vi "TabVisibility.vi"(1 "Page Visible":bool, 2 "array":refnum<vi>[](array[refnum]), 3 "MyfinalExpGraphCont":T1(tab)) -> ()   [LabVIEW 2019]
uses:
  C:/Users/manip/Documents/Controle_Manip_2020/Thorlabs.MotionControl.Controls.dll
  Thorlabs.MotionControl.Controls.dll
  C:/Users/manip/Documents/Controle_Manip_2020/Thorlabs.MotionControl.KCube.SolenoidCLI.dll
  Thorlabs.MotionControl.KCube.SolenoidCLI.dll
  C:/Users/manip/Documents/Controle_Manip_2020/Thorlabs.MotionControl.KCube.PiezoCLI.dll
  Thorlabs.MotionControl.KCube.PiezoCLI.dll
  C:/Program Files/Thorlabs/Scientific Imaging/DCx Camera Support/Develop/DotNet/uc480DotNet.dll
  Program Files/Thorlabs/Scientific Imaging/DCx Camera Support/Develop/DotNet/uc480DotNet.dll
  Light Field/lightfield-automation-labview/LightField Automation.lvclass
  Controls/Control 1.ctl
panel:
  out "Duration 2":dbl caption="s"
  in  "Acquire N: N 2":dbl=10.0 caption="N"
  in  "Acquire Time Trace 2":bool caption="Acquire N"
  in  "CCD 1D Spectrum Main  Cursor2WL 2 Mono 4":bool caption="CCD 1D Spectrum Main  Cursor2WL"
  in  "CCD 1D Spectrum Main  Cursor2WL 1 Mono 4":bool caption="CCD 1D Spectrum Main  Cursor2WL"
  in  "CCD 1D Spectrum Main  Cursor2WL 2 Mono 3":bool caption="CCD 1D Spectrum Main  Cursor2WL"
  in  "CCD 1D Spectrum Main  Cursor2WL 1 Mono 3":bool caption="CCD 1D Spectrum Main  Cursor2WL"
  out "CCD 1D Spectrum Main Cursor 1 nm 2":dbl caption="nm"
  out "CCD 1D Spectrum Main Cursor 2 nm 2":dbl caption="nm"
  in  "Full scale 2":bool
  in  "Acquire Continuous Spectrum 2":bool
  in  "Acquire Spectrum 2":bool
  out "CCD 2D Image Main 2":dbl[][](graph)
  in  "Save Spectrum N 2":bool
  in  "Save Spectrum 2":bool
  out "CCD 1D Spectrum Main 2":T2
  in  "Stop continuous 2":bool
  out "CCD 1D Spectrum Main Energy Scale 2":cluster{dbl[], dbl[]}(graph)
  out "CCD 1D Spectrum Main Cursor 4":dbl caption="eV" format="%#_6p"
  out "CCD 1D Spectrum Main Cursor 3":dbl caption="eV" format="%#_6p"
  out "CCD 1D Spectrum Main deltaE 2":dbl caption="eV" format="%#_3p"
  out "CCD 1D Spectrum Main deltanm 2":dbl caption="m" format="%#_3p"
  in  "Scan FSM Set as Center 2":bool
  in  "Scan FSM Go to Cursor 2":bool
  out "XY Intensity Map 2":dbl[][](graph)
  out "CCD 2D Image XY Map 2":dbl[][](graph)
  out "CCD 1D Spectrum XY Map 2":cluster{dbl[], dbl[]}(graph)
  out "CCD 1D XY Map Spectrum Main Energy Scale 2":cluster{dbl[], dbl[]}(graph)
  in  "NewDot 2":bool caption="NewDot?"
  out "ExportMapPosition? 2":bool caption="Export NC Pos in Map Image?"
  out "Polarisation 2D Image 2":dbl[][](graph)
  out "Polarisation 1D Spectrum 2":cluster{dbl[], dbl[]}(graph) caption="360.0°"
  out "Polarisation 1D Spectrum Energy Scale 2":cluster{dbl[], dbl[]}(graph)
  out "Contrast 2":dbl format="%#_3g"
  out "Contrast Oscillations 2":cluster{dbl[], dbl[]}(graph)
  out "Contrast 1D Spectrum 2":cluster{dbl[], dbl[]}(graph) caption="52924"
  in  "Cursor controls 2":bool
  out "Contrast 1D Spectrum from Cursors 2":cluster{dbl[], dbl[]}(graph) caption="2708"
  in  "Spectrum Custom Continuous Mode 2":u16(ring)=1 caption="Detector(s)" items=["PD", "APD 1", "APD 2", "APD 1+2"]
  in  "Stop PD 2":bool
  in  "Acquire PD 2":bool
  out "PD 1D Spectrum 2":dbl[][](graph)
  in  "PH_SyncDiv 2":enum16{"1", "2", "4", "8"}(ring) caption="SyncDiv"
  in  "PH_CFD0 level 2":i32=50 caption="CFD0" min=0 max=100
  in  "PH_CFD0 zero X 2":i32=10 caption="CFD0 ZeroX"
  in  "PH_CFD1 level 2":i32=50 caption="CFD1" min=0 max=100
  in  "PH_CFD1 zero X 2":i32=10 caption="CFD1 Zero X"
  in  "PH_Range No. 2":i32 caption="Range No."
  in  "V2um 2":dbl=10.0
  in  "Conv/Energy (eV) 2":dbl caption="Energy :" format="%#_6p"
  in  "Conv/Wavelength (nm) 2":dbl caption="Wavelength :"
  in  "Conv/Wavenumber (m-1) 2":dbl caption="Wavenumber :"
  in  "Conv/Time (s) 2":dbl caption="Time :" format="%#_6p"
  in  "ChangeSample 2":bool
  in  "SampleGoal 2":string
  in  "Write to Markdown? 2":bool
  in  "Synthesis/Solvent 2":string(combo)="tol"
  in  "Synthesis/Polymer 2":string(combo)="PS"
  in  "Synthesis/DilutionPolyRatio 2":dbl=1.5
  in  "SampleOf 2":string(combo)="CsPbBr3 NCs"
  in  "Synthesis/Dilution 2":dbl=8000.0
  in  "Synthesis/Name 2":string(combo)="A_FR_210630"
  in  "Mono2 Velocity 2":dbl caption="Veloc." min=0.0 max=20.0 step=0.01
  out "ANC connected 2":bool
  in  "PicoHarp On? 2":bool
  in  "Cryostation On? 2":bool
  in  "Attocubes On? 2":bool
  in  "PZC200 On? 2":bool
  in  "KCube Shutter On? 2":bool
  in  "KCubes Piezo On? 2":bool
  in  "LightField On? 2":bool
  in  "PM16-120 On? 2":bool
  in  "ESP 300 On? 2":bool
  in  "ESP 301 On? 2":bool
  in  "FSM 300 On? 2":bool
  out "Cryo User Stability 2":dbl=450.0 caption="Stability" min=400.0 max=1100.0 step=1.0 format="%#_6p"
  out "Cryo User Temp 2":dbl=450.0 caption="User" min=400.0 max=1100.0 step=1.0
  out "Cryo Sample Stability 2":dbl=450.0 caption="Stability" min=400.0 max=1100.0 step=1.0 format="%#_6p"
  out "Cryo Sample Temp 2":dbl=450.0 caption="Sample" min=400.0 max=1100.0 step=1.0
  out "Cryo Platform Stability 2":dbl=450.0 caption="Stability" min=400.0 max=1100.0 step=1.0 format="%#_6p"
  out "Cryo Platform Temp 2":dbl=450.0 caption="Platform" min=400.0 max=1100.0 step=1.0
  in  "PZC200 COM Port 2":dbl=6.0 caption="COM Port"
  in  "Laser Diode Current Set 2":dbl(slide)=0.02 caption="Power" min=0.02 max=0.061 scale=0.02..0.0605 scale format="%#_3g"
  in  "Laser on? Control 2":bool
  in  "Diode Driver COM 2":refnum<visa-resource-name>="USB0::0x1313::0x804F::M00549740::INSTR"
  in  "Laser Comm On? 2":bool
  in  "ESP300 COM Port 2":refnum<visa-resource-name>="COM4" caption="COM Port"
  in  "Excitation Wavelength (nm) 2":dbl=450.0 caption="Exc WL (nm)" min=400.0 max=1100.0 step=1.0
  out "Photodiode Status 2":bool caption="Status"
  in  "ESP 301 COM Port 2":refnum<visa-resource-name>="ASRL8::INSTR" caption="COM Port"
  in  "FSM Y Axis 2":tag="cDAQ2Mod1/ao1"
  in  "FSM X Axis  2":tag="cDAQ2Mod1/ao2"
  in  "Slit Width (mm) 2":dbl caption="Slit (mm)" min=0.0 max=5.0 step=0.01
  out "Initialise all devices? 2":bool caption="OK"
  in  "TEC Output 2":bool caption="TEC Output"
  out "TEC Temperature 2":dbl caption="TEC Temp" format="%#_4f"
  out "Laser Safety 2":u16(ring)
  in  "LF Visible 2":bool=TRUE caption="LF Visible ?"
  out "PZC200 Instrument Channel 2":string="RS232/10" caption="PZC200 Port"
  out "Cryostation ID 2":refnum<k5>
  out "Serial Number 2":string caption="Serial"
  out "FSM X Task 2":refnum<k21>
  out "FSM Y Task 2":refnum<k21>
  in  "Cryostat 2":enum16{"Montana", "Oxford"}(ring) caption="Cryo :"
  out "CCD T° : 2":dbl
  in  "Synthesis/InjTemp 2":dbl=180.0
  in  "Sample first cooldown 2":timestamp=timestamp(3707971200 s since 1904-01-01) format="%<%x %.3X>T"
  out "PZAPos&Pow 2":dbl[][](array[numeric])
  out "PZC Error 2":errorcluster
  in  "ESP 301 Error 2":errorcluster
  out "KCubeSolenoidControl Reference 2":refnum<k24>
  out "KCube Shutter Device Reference 2":refnum<k24>
  out "KCubePiezoDevice Z Reference 2":refnum<k24>
  out "KCubePiezoControl Z Reference 2":refnum<k24>
  out "KCubePiezoControl Y Reference 2":refnum<k24>
  out "KCubePiezoDevice Y Reference 2":refnum<k24>
  out "KCubePiezoDevice X Reference 2":refnum<k24>
  out "KCubePiezoControl X Reference 2":refnum<k24>
  out "Wavelength calibration 2":dbl[](array[numeric])
  out "Photodiode handle out 2":refnum<visa-resource-name> caption="instrument handle out"
  out "Photodiode error out 2":errorcluster caption="error out" {"code" format="%.0x"}
  out "LightField Automation error out 2":errorcluster
  out "Scan Polar Params 2":refnum<vi>[](array[refnum])
  out "Angles 2":dbl[](array[numeric])
  out "Scan XY Map Params 2":refnum<vi>[](array[refnum])
  out "Thorcam Error 2":errorcluster caption="Error Out"
  out "Data 2":T3(array[cluster])
  in  "ESP300 Error 2":errorcluster
  out "ThorCam Reference 2":refnum<k24>
  out "LightField Automation out 2":refnum<class "LightField Automation.lvclass">
  out "Response 2":string
  out "PZA12 Positions 2":dbl[](array[numeric])
  out "Contrast Array Out 2":dbl[][](array[numeric])
  out "Michelson Array Out 2":dbl[][][](array[numeric])
  out "Pol 2D Array Out 2":dbl[][](array[numeric])
  out "PZC&Pow3D 2":dbl[][][](array[numeric])
  out "Scan Translation Params 2":T4
  out "Scan Contrast Ctrls 2":refnum<vi>[](array[refnum])
  out "ESP Pos 2":dbl[](array[numeric])
  out "ourDLL 2":path
  out "Diode Driver Error out 2":errorcluster
  out "Diode Driver Error 2":errorcluster caption="error in (no error)" {"code" format="%.0x"}
  out "Scan Translation Coarse Ctrls 2":refnum<vi>[](array[refnum])
  out "Scan Spectrum Cust Params 2":refnum<vi>[](array[refnum])
  out "Position (units) 2":dbl format="%.6g"
  out "Att Error 2":errorcluster
  in  "Experiment Graph Controls Tabs":refnum<vi>
  in  "Experiment Graph Controls 2":T5(tab)
  out "Duration":dbl caption="s"
  in  "Acquire N: N":dbl=10.0 caption="N"
  in  "Acquire Time Trace":bool caption="Acquire N"
  in  "CCD 1D Spectrum Main  Cursor2WL 2 Mono 2":bool caption="CCD 1D Spectrum Main  Cursor2WL"
  in  "CCD 1D Spectrum Main  Cursor2WL 1 Mono 2":bool caption="CCD 1D Spectrum Main  Cursor2WL"
  in  "CCD 1D Spectrum Main  Cursor2WL 2 Mono 1":bool caption="CCD 1D Spectrum Main  Cursor2WL"
  in  "CCD 1D Spectrum Main  Cursor2WL 1 Mono 1":bool caption="CCD 1D Spectrum Main  Cursor2WL"
  out "CCD 1D Spectrum Main Cursor 1 nm":dbl caption="nm"
  out "CCD 1D Spectrum Main Cursor 2 nm":dbl caption="nm"
  in  "Full scale":bool
  in  "Acquire Continuous Spectrum":bool
  in  "Acquire Spectrum":bool
  out "CCD 2D Image Main":dbl[][](graph)
  in  "Save Spectrum N":bool
  in  "Save Spectrum":bool
  out "CCD 1D Spectrum Main":T2
  in  "Stop continuous":bool
  out "CCD 1D Spectrum Main Energy Scale":cluster{dbl[], dbl[]}(graph)
  out "CCD 1D Spectrum Main Cursor":dbl caption="eV" format="%#_6p"
  out "CCD 1D Spectrum Main Cursor 2":dbl caption="eV" format="%#_6p"
  out "CCD 1D Spectrum Main deltaE":dbl caption="eV" format="%#_3p"
  out "CCD 1D Spectrum Main deltanm":dbl caption="m" format="%#_3p"
  in  "Scan FSM Set as Center":bool
  in  "Scan FSM Go to Cursor":bool
  out "XY Intensity Map":dbl[][](graph)
  out "CCD 2D Image XY Map":dbl[][](graph)
  out "CCD 1D Spectrum XY Map":cluster{dbl[], dbl[]}(graph)
  out "CCD 1D XY Map Spectrum Main Energy Scale":cluster{dbl[], dbl[]}(graph)
  in  "NewDot":bool caption="NewDot?"
  out "ExportMapPosition?":bool caption="Export NC Pos in Map Image?"
  out "Polarisation 2D Image":dbl[][](graph)
  out "Polarisation 1D Spectrum":cluster{dbl[], dbl[]}(graph) caption="360.0°"
  out "Polarisation 1D Spectrum Energy Scale":cluster{dbl[], dbl[]}(graph)
  out "Contrast":dbl format="%#_3g"
  out "Contrast Oscillations":cluster{dbl[], dbl[]}(graph)
  out "Contrast 1D Spectrum":cluster{dbl[], dbl[]}(graph) caption="52924"
  in  "Cursor controls":bool
  out "Contrast 1D Spectrum from Cursors":cluster{dbl[], dbl[]}(graph) caption="2708"
  in  "Spectrum Custom Continuous Mode":u16(ring)=1 caption="Detector(s)" items=["PD", "APD 1", "APD 2", "APD 1+2"]
  in  "Stop PD":bool
  in  "Acquire PD":bool
  out "PD 1D Spectrum":dbl[][](graph)
  in  "PH_SyncDiv":enum16{"1", "2", "4", "8"}(ring) caption="SyncDiv"
  in  "PH_CFD0 level":i32=50 caption="CFD0" min=0 max=100
  in  "PH_CFD0 zero X":i32=10 caption="CFD0 ZeroX"
  in  "PH_CFD1 level":i32=50 caption="CFD1" min=0 max=100
  in  "PH_CFD1 zero X":i32=10 caption="CFD1 Zero X"
  in  "PH_Range No.":i32 caption="Range No."
  in  "V2um":dbl=10.0
  in  "Conv/Energy (eV)":dbl caption="Energy :" format="%#_6p"
  in  "Conv/Wavelength (nm)":dbl caption="Wavelength :"
  in  "Conv/Wavenumber (m-1)":dbl caption="Wavenumber :"
  in  "Conv/Time (s)":dbl caption="Time :" format="%#_6p"
  in  "ChangeSample":bool
  in  "SampleGoal":string
  in  "Write to Markdown?":bool
  in  "Synthesis/Solvent":string(combo)="tol"
  in  "Synthesis/Polymer":string(combo)="PS"
  in  "Synthesis/DilutionPolyRatio":dbl=1.5
  in  "SampleOf":string(combo)="CsPbBr3 NCs"
  in  "Synthesis/Dilution":dbl=8000.0
  in  "Synthesis/Name":string(combo)="A_FR_210630"
  in  "Mono2 Velocity":dbl caption="Veloc." min=0.0 max=20.0 step=0.01
  out "ANC connected":bool
  in  "PicoHarp On?":bool
  in  "Cryostation On?":bool
  in  "Attocubes On?":bool
  in  "PZC200 On?":bool
  in  "KCube Shutter On?":bool
  in  "KCubes Piezo On?":bool
  in  "LightField On?":bool
  in  "PM16-120 On?":bool
  in  "ESP 300 On?":bool
  in  "ESP 301 On?":bool
  in  "FSM 300 On?":bool
  out "Cryo User Stability":dbl=450.0 caption="Stability" min=400.0 max=1100.0 step=1.0 format="%#_6p"
  out "Cryo User Temp":dbl=450.0 caption="User" min=400.0 max=1100.0 step=1.0
  out "Cryo Sample Stability":dbl=450.0 caption="Stability" min=400.0 max=1100.0 step=1.0 format="%#_6p"
  out "Cryo Sample Temp":dbl=450.0 caption="Sample" min=400.0 max=1100.0 step=1.0
  out "Cryo Platform Stability":dbl=450.0 caption="Stability" min=400.0 max=1100.0 step=1.0 format="%#_6p"
  out "Cryo Platform Temp":dbl=450.0 caption="Platform" min=400.0 max=1100.0 step=1.0
  in  "PZC200 COM Port":dbl=6.0 caption="COM Port"
  in  "Laser Diode Current Set":dbl(slide)=0.02 caption="Power" min=0.02 max=0.061 scale=0.02..0.0605 scale format="%#_3g"
  in  "Laser on? Control":bool
  in  "Diode Driver COM":refnum<visa-resource-name>="USB0::0x1313::0x804F::M00549740::INSTR"
  in  "Laser Comm On?":bool
  in  "ESP300 COM Port":refnum<visa-resource-name>="COM4" caption="COM Port"
  in  "Excitation Wavelength (nm)":dbl=450.0 caption="Exc WL (nm)" min=400.0 max=1100.0 step=1.0
  out "Photodiode Status":bool caption="Status"
  in  "ESP 301 COM Port":refnum<visa-resource-name>="ASRL8::INSTR" caption="COM Port"
  in  "FSM Y Axis":tag="cDAQ2Mod1/ao1"
  in  "FSM X Axis":tag="cDAQ2Mod1/ao2"
  in  "Slit Width (mm)":dbl caption="Slit (mm)" min=0.0 max=5.0 step=0.01
  out "Initialise all devices?":bool caption="OK"
  in  "TEC Output":bool
  out "TEC Temperature":dbl caption="TEC Temp" format="%#_4f"
  out "Laser Safety":u16(ring)
  in  "LF Visible":bool=TRUE caption="LF Visible ?"
  out "PZC200 Instrument Channel":string="RS232/10" caption="PZC200 Port"
  out "Cryostation ID":refnum<k5>
  out "Serial Number":string caption="Serial"
  out "FSM X Task":refnum<k21>
  out "FSM Y Task":refnum<k21>
  in  "Cryostat":enum16{"Montana", "Oxford"}(ring) caption="Cryo :"
  out "CCD T° :":dbl
  in  "Synthesis/InjTemp":dbl=180.0
  in  "Sample first cooldown":timestamp=timestamp(3707971200 s since 1904-01-01) format="%<%x %.3X>T"
  out "PZAPos&Pow":dbl[][](array[numeric])
  out "PZC Error":errorcluster
  in  "ESP 301 Error":errorcluster
  out "KCubeSolenoidControl Reference":refnum<k24>
  out "KCube Shutter Device Reference":refnum<k24>
  out "KCubePiezoDevice Z Reference":refnum<k24>
  out "KCubePiezoControl Z Reference":refnum<k24>
  out "KCubePiezoControl Y Reference":refnum<k24>
  out "KCubePiezoDevice Y Reference":refnum<k24>
  out "KCubePiezoDevice X Reference":refnum<k24>
  out "KCubePiezoControl X Reference":refnum<k24>
  out "Wavelength calibration":dbl[](array[numeric])
  out "Photodiode handle out":refnum<visa-resource-name> caption="instrument handle out"
  out "Photodiode error out":errorcluster caption="error out" {"code" format="%.0x"}
  out "LightField Automation error out":errorcluster
  out "Scan Polar Params":refnum<vi>[](array[refnum])
  out "Angles":dbl[](array[numeric])
  out "Scan XY Map Params":refnum<vi>[](array[refnum])
  out "Thorcam Error":errorcluster caption="Error Out"
  out "Data":T3(array[cluster])
  in  "ESP300 Error":errorcluster
  out "ThorCam Reference":refnum<k24>
  out "LightField Automation out":refnum<class "LightField Automation.lvclass">
  out "Response":string
  out "PZA12 Positions":dbl[](array[numeric])
  out "Contrast Array Out":dbl[][](array[numeric])
  out "Michelson Array Out":dbl[][][](array[numeric])
  out "Pol 2D Array Out":dbl[][](array[numeric])
  out "PZC&Pow3D":dbl[][][](array[numeric])
  out "Scan Translation Params":T4
  out "Scan Contrast Ctrls":refnum<vi>[](array[refnum])
  out "ESP Pos":dbl[](array[numeric])
  out "ourDLL":path
  out "Diode Driver Error out":errorcluster
  out "Diode Driver Error":errorcluster caption="error in (no error)" {"code" format="%.0x"}
  out "Scan Translation Coarse Ctrls":refnum<vi>[](array[refnum])
  out "Scan Spectrum Cust Params":refnum<vi>[](array[refnum])
  out "Position (units)":dbl format="%.6g"
  out "Att Error":errorcluster
  in  "Experiment Graph Controls":T5(ring)=enum."Settings"
  # "Mono 1"
  # "Mono 2"
  # "--|--"
  # "Acquisition"
  # "CenterWL"
  # "l   ="
  # "E  ="
  # "DE ="
  # "1"
  # "1"
  # "--|--"
  # "Dl ="
  # "f(time)"
  # "CenterWL"
  # "l   ="
  # "E   ="
  # "2"
  # "2"
  # "and increment NC number"
  # "CFD"
  # "Zero Cross"
  # "Sync/CH0"
  # "CFD"
  # "CH1"
  # "Zero Cross"
  # "Absolute conversions"
  # "change one value manually and the others will update accordingly"
  # "Detection efficiency"
  # "For the steering mirror, in the current configuration 1 V equals to                um."
  # "eV"
  # "nm"
  # "-1"
  # "cm"
  # "s"
  # "Thorlabs Laser Diode Driver CLD1010"
  # "min"
  # "max"
  # "Newport FSM-300-01"
  # "Newport ESP 301"
  # "Axis 2: Det"
  # "Axis 3: Exc"
  # "Axis 1"
  # "Montana Cryostation s50"
  # "Newport PZC200"
  # "Thorlabs Shutter SH05"
  # "Thorlabs NanoMax + 3 Axis Piezos"
  # "Attocube ANC350 - 2 ANPx51 & 1 ANPz51"
  # "Synthesis and sample details"
  # "Inside the cryostat, there is a sample of"
  # "Newport ESP 300"
  # "The sample currently inside the cryostat is from the                                 synthesis made"
  # "with an injection temperature of          °C.  The sample was prepared by dispersing"
  # "a solution diluted                     times in a          % solution of                               in                        ."
  # "The sample was prepared on"
  # "PicoHarp 300"
  # "Thorlabs PM16-120"
  # "Princeton HRS-500 + Pixis"
  # "The sample is inside the cryostat in order to:"
  # "°C"
  # "Mono 1"
  # "Mono 2"
  # "--|--"
  # "Acquisition"
  # "CenterWL"
  # "l   ="
  # "E  ="
  # "DE ="
  # "1"
  # "1"
  # "--|--"
  # "Dl ="
  # "f(time)"
  # "CenterWL"
  # "l   ="
  # "E   ="
  # "2"
  # "2"
  # "and increment NC number"
  # "CFD"
  # "Zero Cross"
  # "Sync/CH0"
  # "CFD"
  # "CH1"
  # "Zero Cross"
  # "Absolute conversions"
  # "change one value manually and the others will update accordingly"
  # "Detection efficiency"
  # "For the steering mirror, in the current configuration 1 V equals to                um."
  # "eV"
  # "nm"
  # "-1"
  # "cm"
  # "s"
  # "Thorlabs Laser Diode Driver CLD1010"
  # "min"
  # "max"
  # "Newport FSM-300-01"
  # "Newport ESP 301"
  # "Axis 2: Det"
  # "Axis 3: Exc"
  # "Axis 1"
  # "Montana Cryostation s50"
  # "Newport PZC200"
  # "Thorlabs Shutter SH05"
  # "Thorlabs NanoMax + 3 Axis Piezos"
  # "Attocube ANC350 - 2 ANPx51 & 1 ANPz51"
  # "Synthesis and sample details"
  # "Inside the cryostat, there is a sample of"
  # "Newport ESP 300"
  # "The sample currently inside the cryostat is from the                                 synthesis made"
  # "with an injection temperature of          °C.  The sample was prepared by dispersing"
  # "a solution diluted                     times in a          % solution of                               in                        ."
  # "The sample was prepared on"
  # "PicoHarp 300"
  # "Thorlabs PM16-120"
  # "Princeton HRS-500 + Pixis"
  # "The sample is inside the cryostat in order to:"
  # "°C"
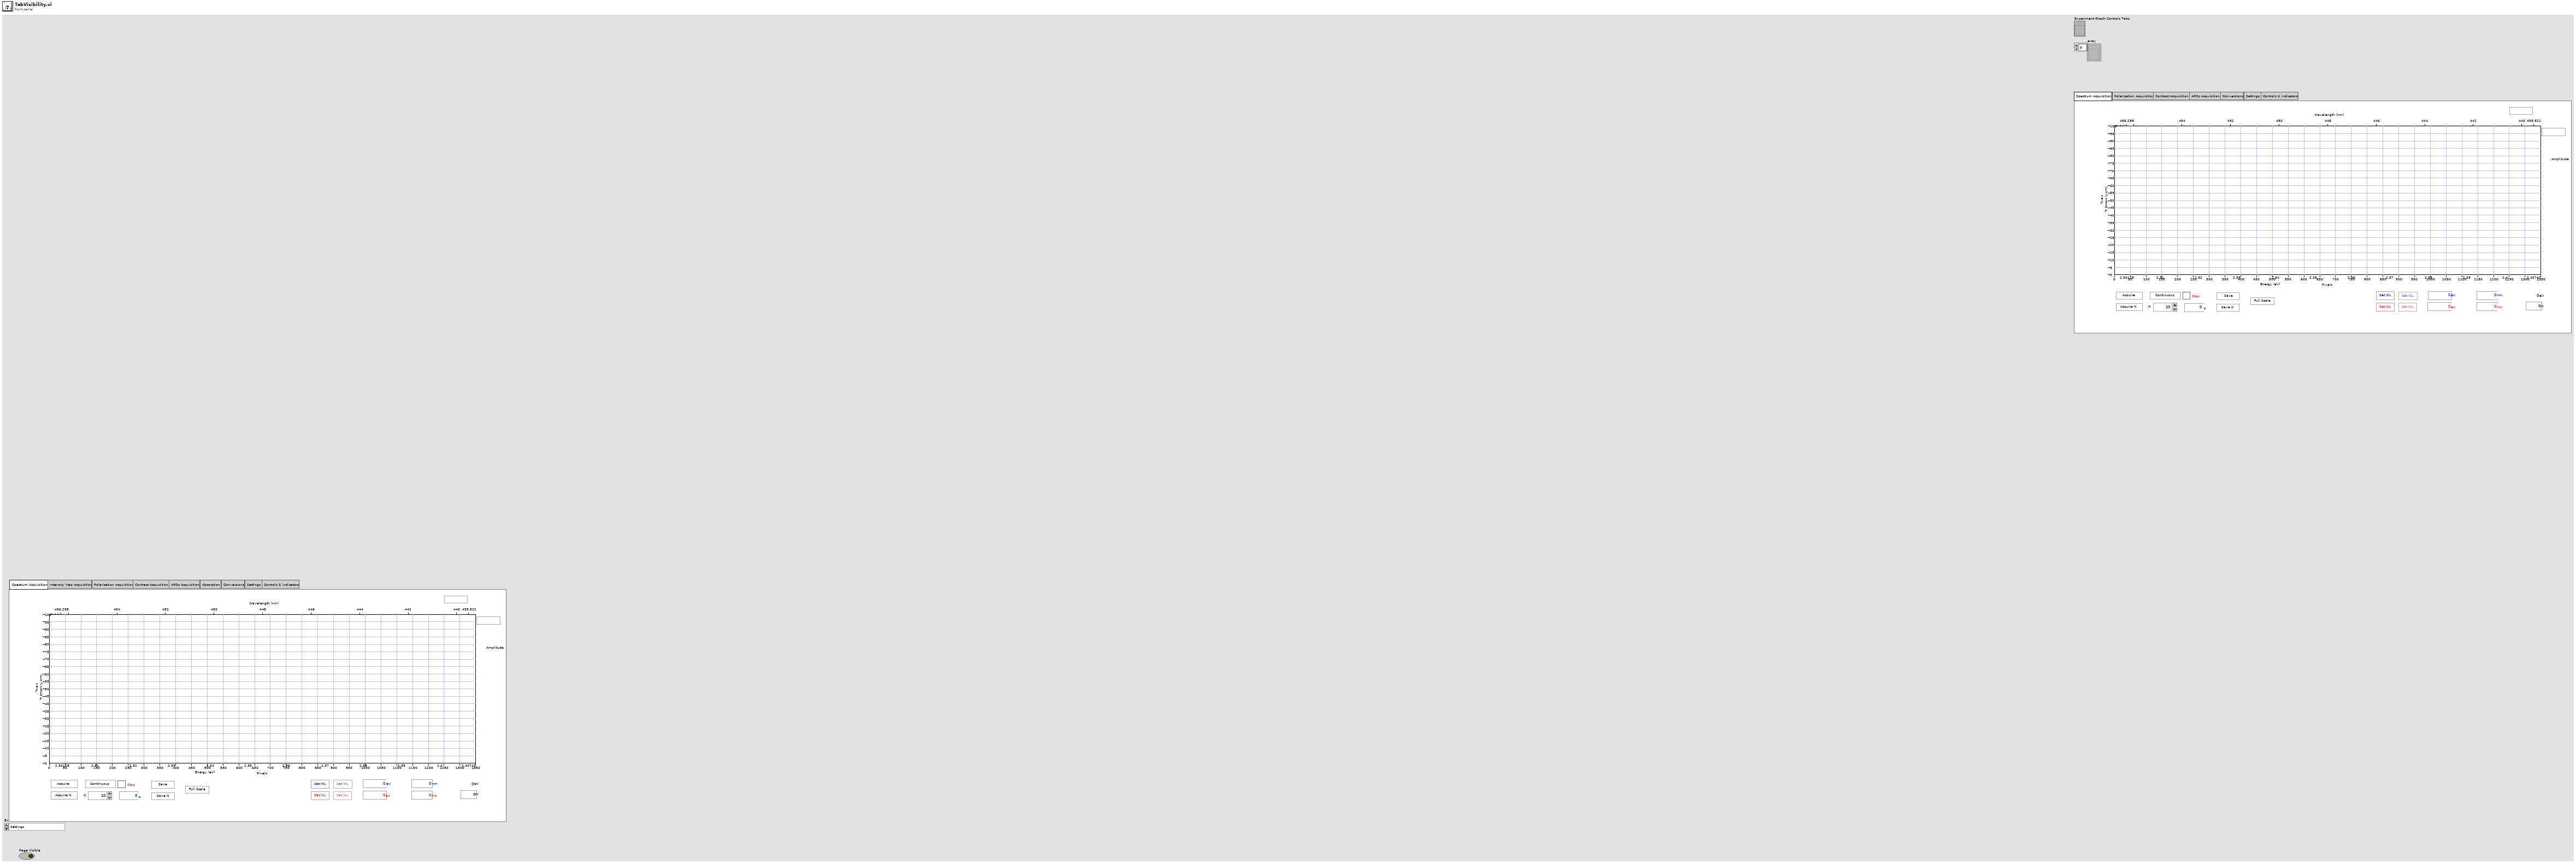
[diagram p1: front panel]
types:
  T1 = enum32{"Spectrum Acquisition", "Intensity Map Acquisition", "Polarisation Acquisition", "Contrast Acquisition", "APDs Acquisition", "Absorption", "Conversions", "Settings", "Controls & indicators"}
  T2 = typedef "Control 1.ctl" = cluster{dbl[], dbl[]}
  T3 = cluster{"Image":dbl[][][], "Frame Size":cluster{"F":i32, "Y":i32, "X":i32}}[]
  T4 = cluster{"LinT Start Pos (mm)":dbl, "LinT Step Pos (mm)":dbl, "LinT End pos (mm)":dbl, "LinTFine Start Pos (usteps)":dbl, "LinTFines Step Pos (usteps)":dbl, "LinTFine End Pos (usteps)":dbl}
  T5 = enum32{"Spectrum Acquisition", "Intensity Map Acquisition", "Polarisation Acquisition", "Contrast Acquisition", "APDs Acquisition", "Conversions", "Settings", "Controls & indicators"}
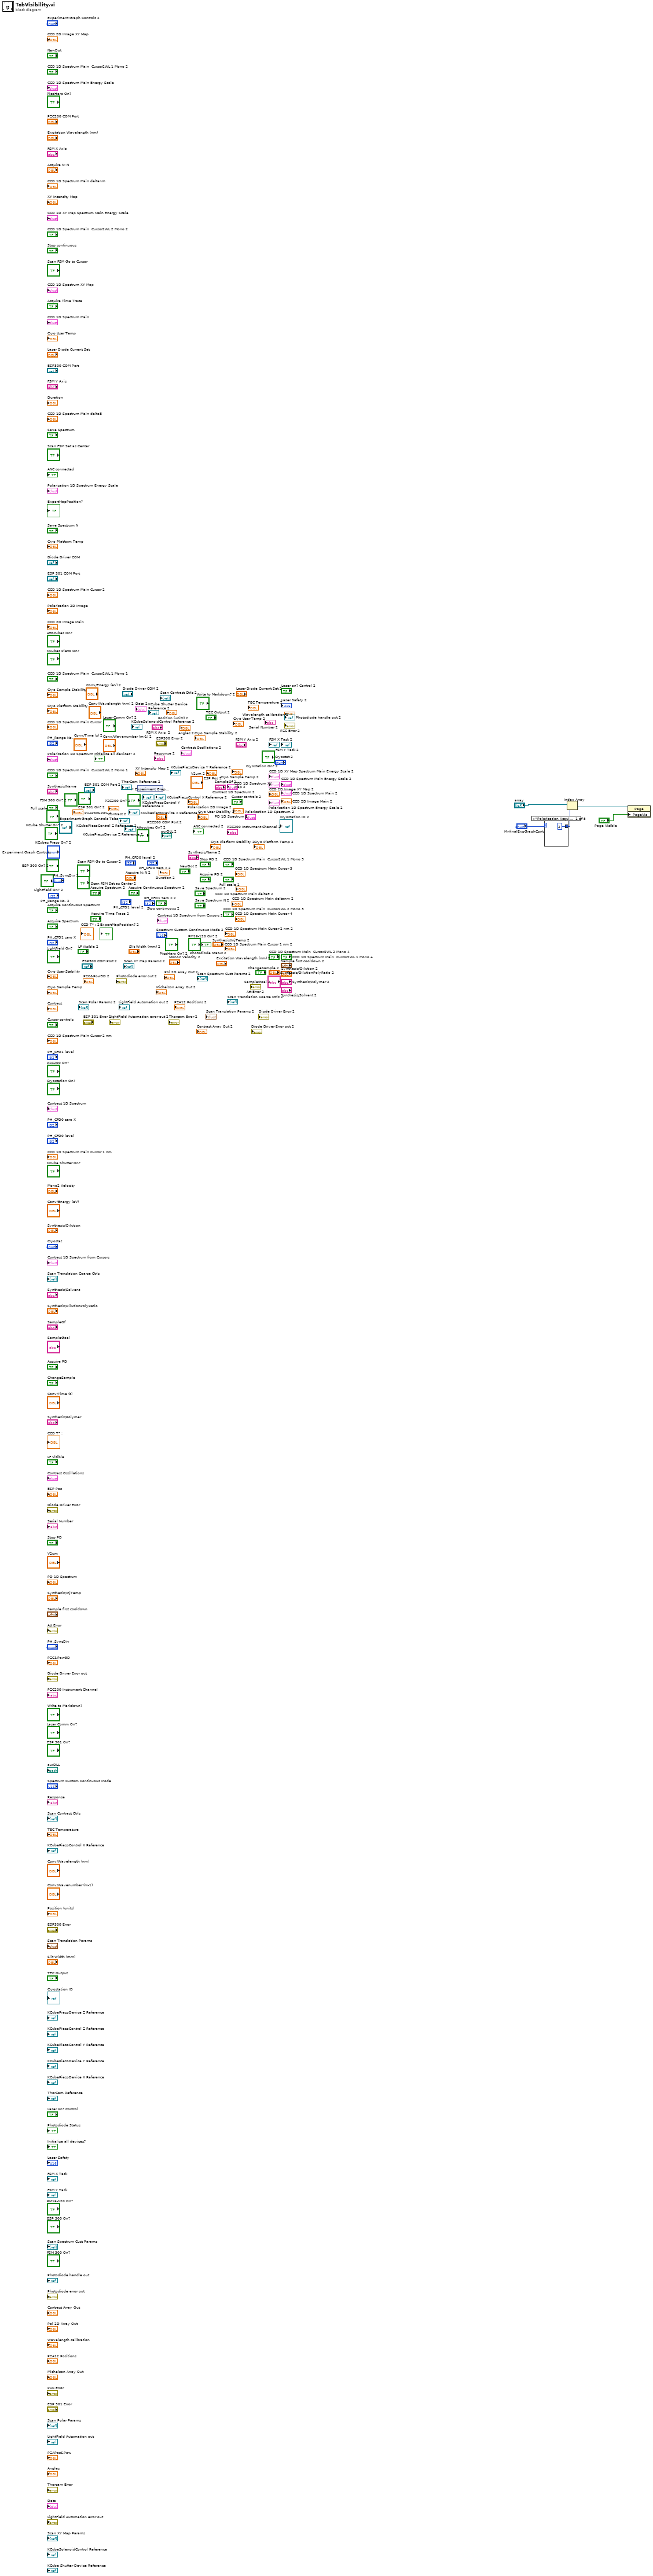
[diagram p0: block diagram]
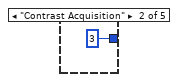
[diagram p2: hidden frame]
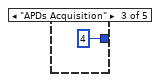
[diagram p3: hidden frame]
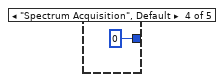
[diagram p4: hidden frame]
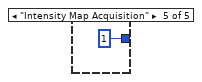
[diagram p5: hidden frame]
diagram:
  n1 = control-ref of="Experiment Graph Controls 2"() -> ()  [unwired: 1 out]
  n2 = case shown="\"Polarisation Acquisition\"" "MyfinalExpGraphCont" {
    tunnel: [2 3 4 0 1] -> w5
    frame "Polarisation Acquisition" {
    }
    frame "Contrast Acquisition" {
    }
    frame "APDs Acquisition" {
    }
    frame "Spectrum Acquisition", Default {
    }
    frame "Intensity Map Acquisition" {
    }
  }
  n3 = Index Array(array="array", index=w5) -> (element=w4:refnum<vi>)
  n4 = property class="Page"(reference=w4, "PageVis"="Page Visible") -> ()  [unwired: 1 in, 2 out]
